vi "Advanced Cut - Main - Copy.vi"   [LabVIEW 2016] (continued)
"Desaccade"=FALSE, "Offset"=0.0, "Gain"=1.0}, {"Color"=16777224, "Visible"=TRUE, "Channel"=13, "Invert"=FALSE, "Desaccade"=FALSE, "Offset"=0.0, "Gain"=1.0}, {"Color"=16777224, "Visible"=FALSE, "Channel"=14, "Invert"=FALSE, "Desaccade"=FALSE, "Offset"=0.0, "Gain"=1.0}, {"Color"=16777224, "Visible"=FALSE, "Channel"=15, "Invert"=FALSE, "Desaccade"=FALSE, "Offset"=0.0, "Gain"=1.0}], "Experiment Parameters"={"Freq"=0.0, "Vel"=0, "Acc"=0, "Stimulus"="Head Impulse"}, "Autosort File"=refnum, "Data File"={"Data Channels"=array34x71049[2415666 elements], "Sample Rate"=500, "Channel List"=["Hz Position-in-Head", "Hz Velocity-in-Head", "Hy Position-in-Head", "Hy Velocity-in-Head", "Hx Position-in-Head", "Hx Velocity-in-Head", "Hl Velocity-in-Head", "Hr Velocity-in-Head", "Lx Position-in-Head", "Ly Position-in-Head", "Lz Position-in-Head", "Lx Velocity-in-Head", "Ly Velocity-in-Head", "Lz Velocity-in-Head", "Ll Velocity-in-Head", "Lr Velocity-in-Head", "Rx Position-in-Head", "Ry Position-in-Head", "Rz Position-in-Head", "Rx Velocity-in-Head", "Ry Velocity-in-Head", "Rz Velocity-in-Head", "Rl Velocity-in-Head", "Rr Velocity-in-Head", "Target on/off", "aux input 1", "aux input 2", " ", "", "", "", "Target Hor", "Target Ver", ""]}, "Experiment data path"=path "C:/Users/w.figtree/Desktop/Coils Data/3", "Image data path"=path "/Macintosh HD/Users/patrick/Studium/Diploma Thesis/Data Analysis", "LVS data path"=path "/Macintosh HD/Users/patrick/Studium/Diploma Thesis/Data Analysis", "Raw copy path"=path "/Macintosh HD/Users/patrick/Studium/Diploma Thesis/Data Analysis", "filename"="passive_lvs.lvs", "desaccading parameters"={"Tolerance"=3, "Acc Range"=7000.0, "Sample Rate"=500, "Impulse Plane 2"=enum."Yaw", "Impulse dir"=FALSE}, "Experiment Parameters 2"={"Subject"="SE Trial Short Term", "Strain"="", "Rotation plane"="", "Experimenter"=" ", "Trial"=0.0, "Time"=0.0}, "Excel"={"Excel._Application"=refnum, "Use Excel"=TRUE, "Worksheet SINE"=refnum, "Row SINE"=0, "Worksheet TRANS"=refnum, "Row TRANS"=0}, "Session Config File"=refnum, "Autosort Parameter Set"=4, "EMA Version"="EMA 2016a", "desacc "={"Threshold 1 [Acc]"=7000.0, "Threshold 2 [% of TH1]"=60, "tolerance"=3, "Search WD "=0.1, " always use TH2"=FALSE, "Range"=3.0, "Max time"=120.0, "Min time"=20.0, "Velocity Threshold"=150}, "Cycle Nr for Saccades"={"POS"=0, "NEG"=0}, "Undo Counter"=0, "History Length"=0, "Redo Counter"=0, "Histpry Position"=-1, "Raw Data File"={"Data Channels"=[], "Sample Rate"=0, "Channel List"=[]}, "calibration name"="u_calibration_1_p00001s001_calib.mat"} {"Parameter Time Series"."time offset" format="%.3f"; "Parameter Time Series"."Gain" format="%.1f"; "Parameter Time Series"."Offset" format="%.1f"; "Parameter Time Series"."List 1" items=["Motor-Pos", "Motor-Vel", "Lx Position-in-Head", "Ly Position-in-Head", "Lz Position-in-Head", "Lx Velocity-in-Head", "Ly Velocity-in-Head", "Lz Velocity-in-Head", "Ll Velocity-in-Head", "Lr Velocity-in-Head", "Lx Accel-in-Head", "Ly Accel-in-Head", "Lz Accel-in-Head", "Rx Position-in-Head", "Ry Position-in-Head", "Rz Position-in-Head", "Rx Velocity-in-Head", "Ry Velocity-in-Head", "Rz Velocity-in-Head", "Rl Velocity-in-Head", "Rr Velocity-in-Head", "Rx Accel-in-Head", "Ry Accel-in-Head", "Rz Accel-in-Head", "Global Trigger", "", "", ""]; "Parameter Impuls Series"."Gain" format="%.1f"; "Parameter Impuls Series"."Offset" format="%.1f"})   [LabVIEW 2016]
uses:
  Type Definitions/Advanced Cut States.ctl
  Type Definitions/Snippet.ctl
  <userlib>/_OpenG.lib/file/file.llb/Strip Path Extension - Path__ogtk.vi
  core/type-defs/TD_Impulse Parameter.ctl
  core/core.lvlib
  core/type-defs/TD_Time Series.ctl
  core/type-defs/TD_Statemachine-Data.ctl
panel:
  out "Time Series Graph":cluster{"Ramp Pattern":dbl[], dbl[]}[](graph)
  in  "Snippet File Suffix":string
  in  "btn_DoCut":bool
  in  "btn_AutoSnippet":bool
  in  "btn_ClearTable":bool
  in  "Auto Snippet Options":T1
  in  "Snippet Table":string[][](table)
  in  "Parameter Time Series":T5(array[cluster]) caption="X-off    Y-off     Gain   Inv Filt Dot Int                      Channel                                  Vis" {"time offset" format="%.3f"; "Gain" format="%.1f"; "Offset" format="%.1f"; "List 1" items=["-", "Hz Velocity-in-Head", "-", "Hy Velocity-in-Head", "-", "Hx Velocity-in-Head", "Hl Velocity-in-Head", "Hr Velocity-in-Head", "-", "Ly Position-in-Head", "Lz Position-in-Head", "-", "Ly Velocity-in-Head", "Lz Velocity-in-Head", "-", "-", "-", "-", "-", "-", "-", "-", "-", "-"]}
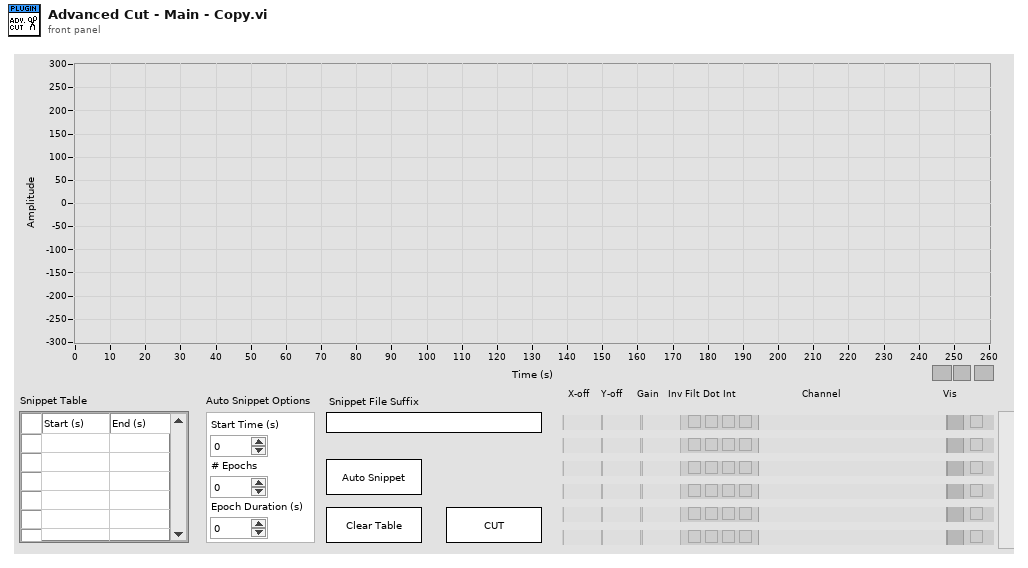
[diagram p1: front panel]
types:
  T1 = cluster{"Start Time (s)":dbl, "# Epochs":u32, "Epoch Duration (s)":dbl}
  T2 = typedef "core.lvlib/TD_Statemachine-Data.ctl" = cluster{"Impulse Positions":cluster{"Start":i32, "End":i32, "Impulse Plane":enum16{"Other", "Yaw", "Pitch", "Roll", "LARP", "RALP"}, "Impulse Direction +ve?":bool, "Time offset":i32, "Amplitude offset":dbl}[], "Old Impulse positions for Undo":cluster{"Start":i32, "End":i32, "Impulse Plane":enum16{"Other", "Yaw", "Pitch", "Roll", "LARP", "RALP"}, "Impulse Direction +ve?":bool, "Time offset":i32, "Amplitude offset":dbl}[][], "No. Imp":i32, "Parameter Time Series":T3, "Parameter Impuls Series":T4, "Experiment Parameters":cluster{"Freq":dbl, "Vel":i32, "Acc":i32, "Stimulus":string}, "Autosort File":refnum<file>, "Data File":cluster{"Data Channels":dbl[][], "Sample Rate":i32, "Channel List":string[]}, "Experiment data path":path, "Image data path":path, "LVS data path":path, "Raw copy path":path, "filename":string, "desaccading parameters":cluster{"Tolerance":i32, "Acc Range":dbl, "Sample Rate":i32, "Impulse Plane 2":enum16{"Other", "Yaw", "Pitch", "Roll", "LARP", "RALP"}, "Impulse dir":bool}, "Experiment Parameters 2":cluster{"Subject":string, "Strain":string, "Rotation plane":string, "Experimenter":string, "Trial":dbl, "Time":dbl}, "Excel":cluster{"Excel._Application":refnum<k7>, "Use Excel":bool, "Worksheet SINE":refnum<k7>, "Row SINE":i32, "Worksheet TRANS":refnum<k7>, "Row TRANS":i32}, "Session Config File":refnum<file>, "Autosort Parameter Set":i32, "EMA Version":string, "desacc ":cluster{"Threshold 1 [Acc]":dbl, "Threshold 2 [% of TH1]":i32, "tolerance":i32, "Search WD ":dbl, " always use TH2":bool, "Range":dbl, "Max time":dbl, "Min time":dbl, "Velocity Threshold":i32}, "Cycle Nr for Saccades":cluster{"POS":i32, "NEG":i32}, "Undo Counter":i32, "History Length":i32, "Redo Counter":i32, "Histpry Position":i32, "Raw Data File":cluster{"Data Channels":dbl[][], "Sample Rate":i32, "Channel List":string[]}, "calibration name":string}
  T3 = typedef "core.lvlib/TD_Time Series.ctl" = cluster{"time offset":dbl, "Offset":dbl, "Gain":dbl, "inverse":bool, "filter data":bool, "dots":bool, "interpolate":bool, "List 1":u16, "Color Box":u32, "Boolean":bool}[]
  T4 = typedef "core.lvlib/TD_Impulse Parameter.ctl" = cluster{"Color":u32, "Visible":bool, "Channel":u16, "Invert":bool, "Desaccade":bool, "Offset":dbl, "Gain":dbl}[]
  T5 = cluster{"time offset":dbl, "Offset":dbl, "Gain":dbl, "inverse":bool, "filter data":bool, "dots":bool, "interpolate":bool, "List 1":u16, "Color Box":u32, "Boolean":bool}[]
  T6 = typedef "Snippet.ctl" = cluster{"Start Index":i32, "End Index":i32}
  T7 = typedef "Advanced Cut States.ctl" = enum16{"Initialise", "Quit", "DO Refresh Snippet Table", "DO Auto Snippet", "DO Clear Snippets", "DO Cut"}
  T8 = typedef "Advanced Cut States.ctl" = enum16{"Initialise", "Quit", "DO Draw", "Draw - Defer Updates", "Draw - Clear Time Series", "Draw - Time Series", "Draw - Snippet Table", "Draw - Enable Updates", "DO Auto Snippet", "DO Clear Snippets", "DO Cut"}
  T9 = cluster{"Data Channels":dbl[][], "Sample Rate":i32, "Channel List":string[]}
  T10 = cluster{"Data File":cluster{"Data Channels":dbl[][], "Sample Rate":i32, "Channel List":string[]}, "Data IN":T2}
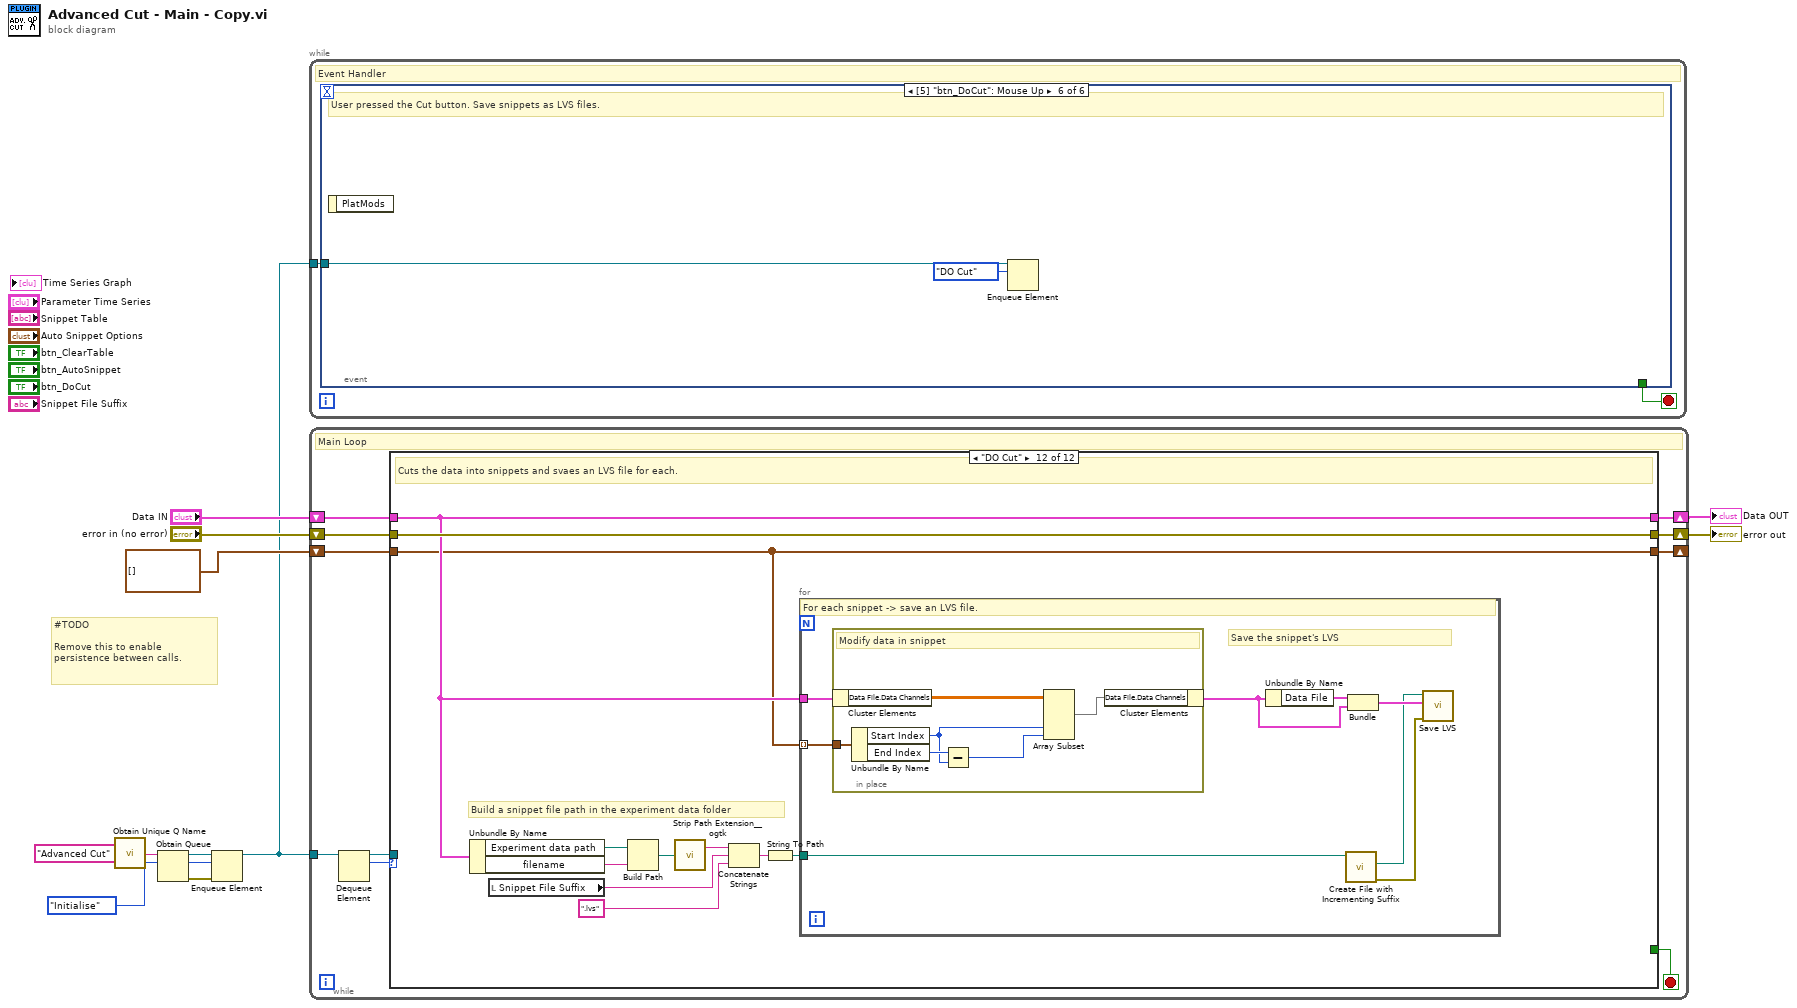
[diagram p0: block diagram]
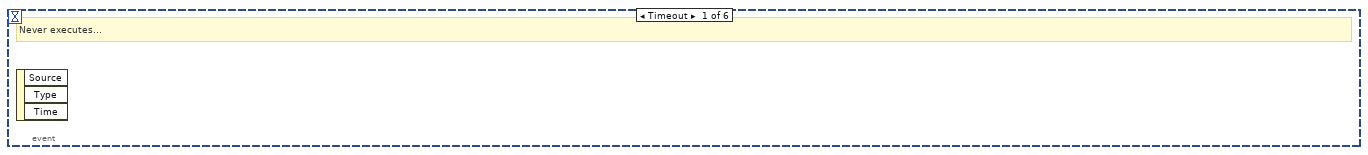
[diagram p2: hidden frame]
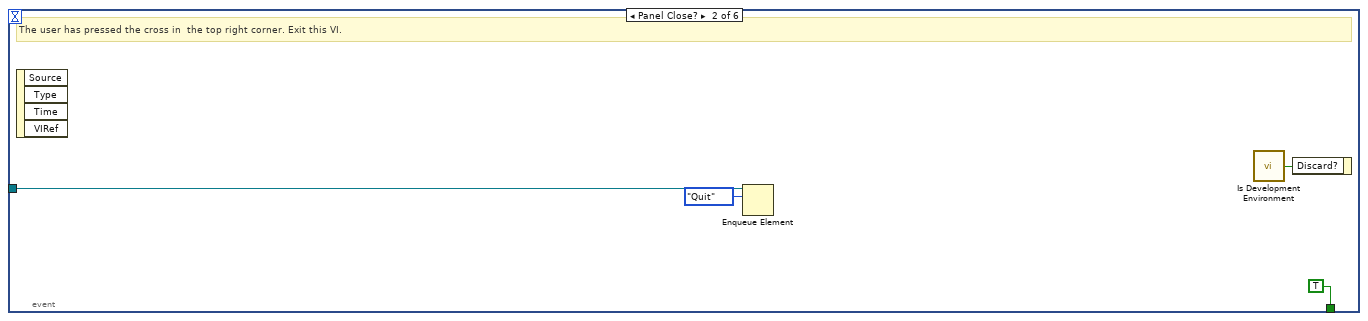
[diagram p3: hidden frame]
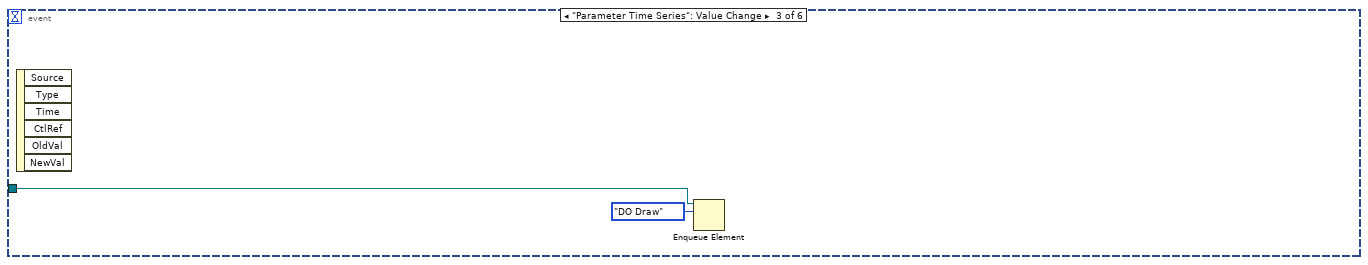
[diagram p4: hidden frame]
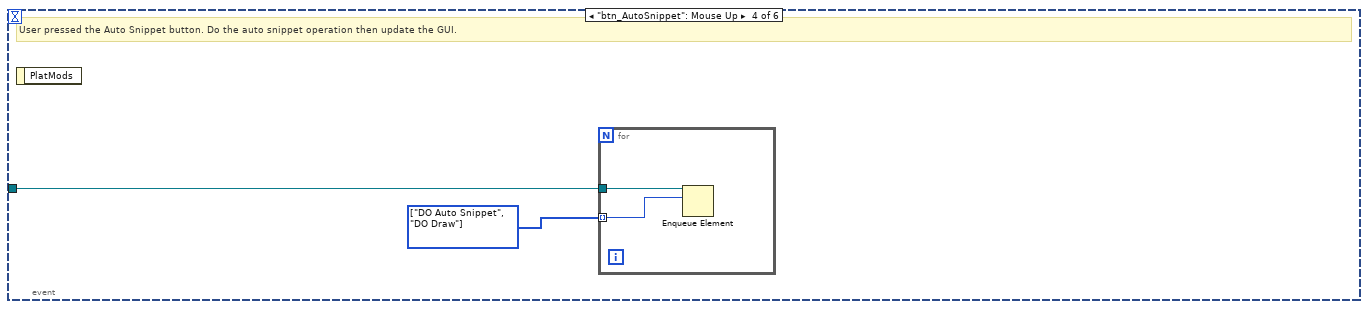
[diagram p5: hidden frame]
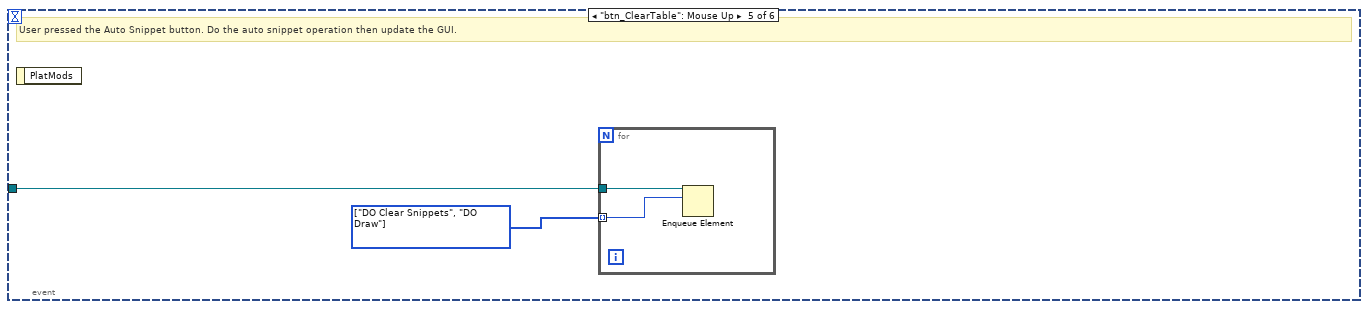
[diagram p6: hidden frame]
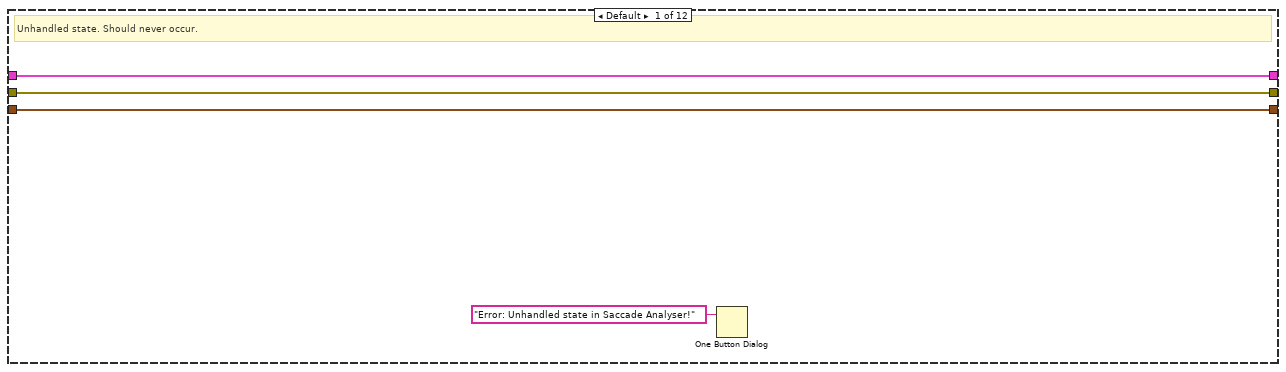
[diagram p7: hidden frame]
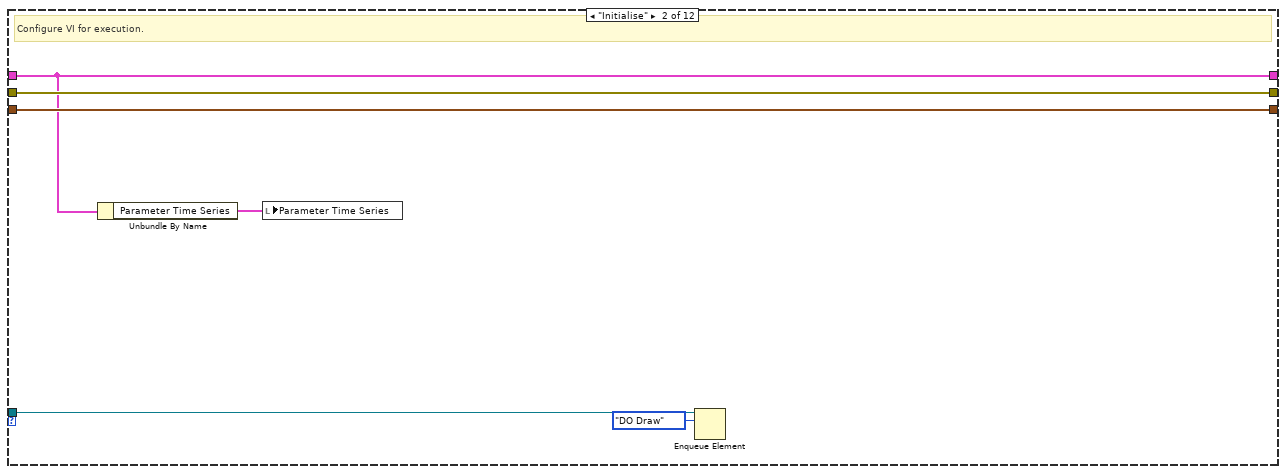
[diagram p8: hidden frame]
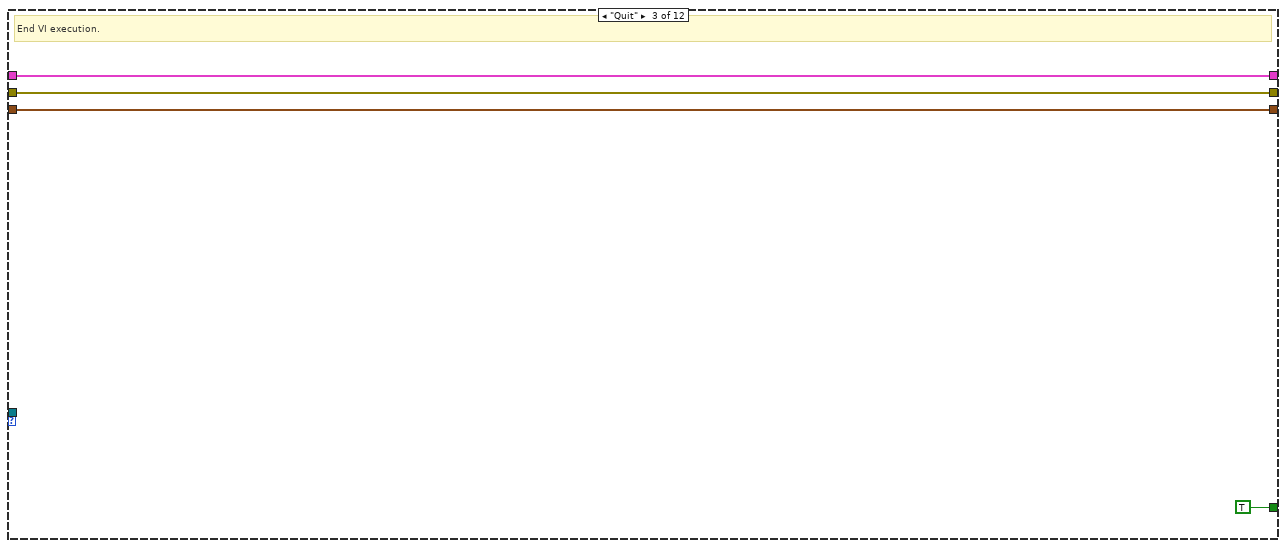
[diagram p9: hidden frame]
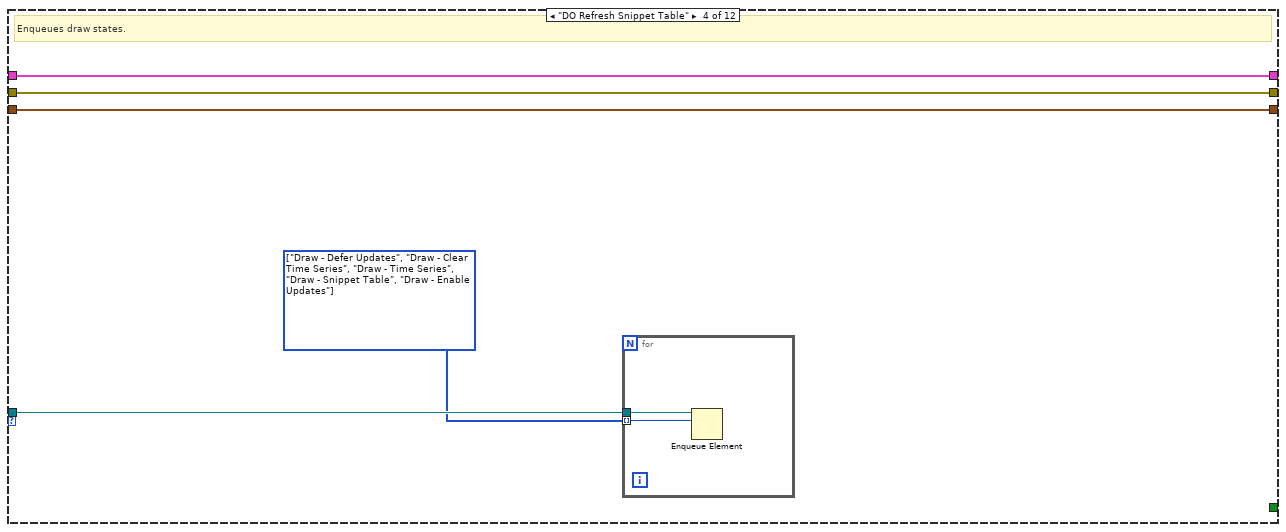
[diagram p10: hidden frame]
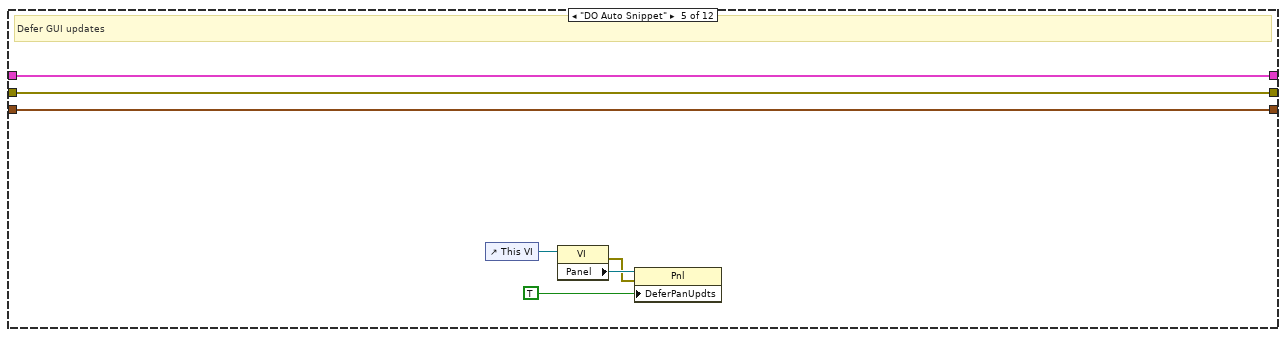
[diagram p11: hidden frame]
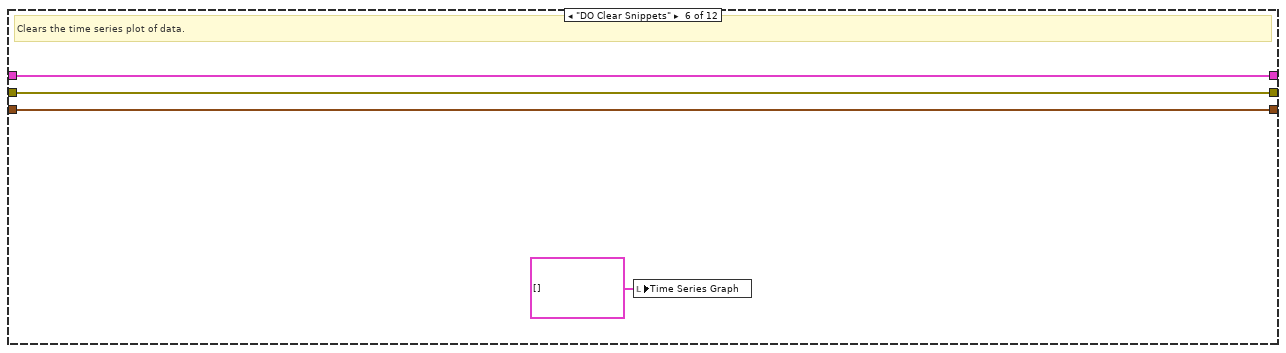
[diagram p12: hidden frame]
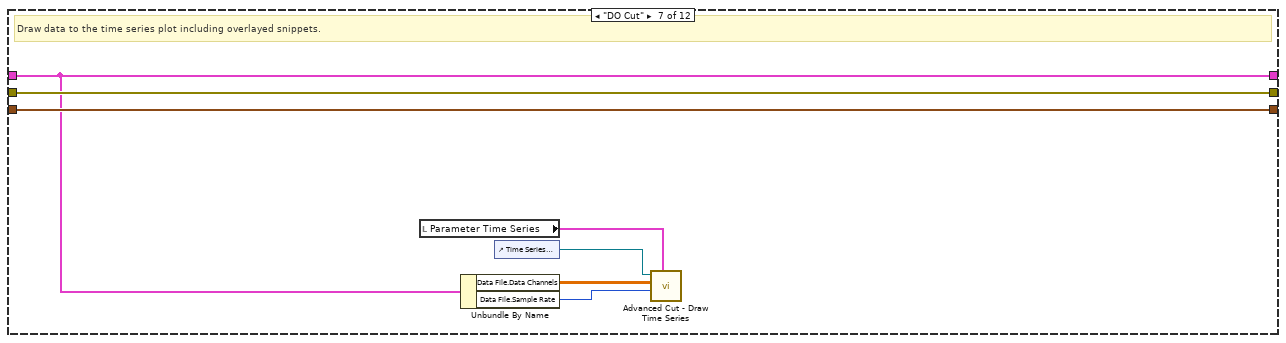
[diagram p13: hidden frame]
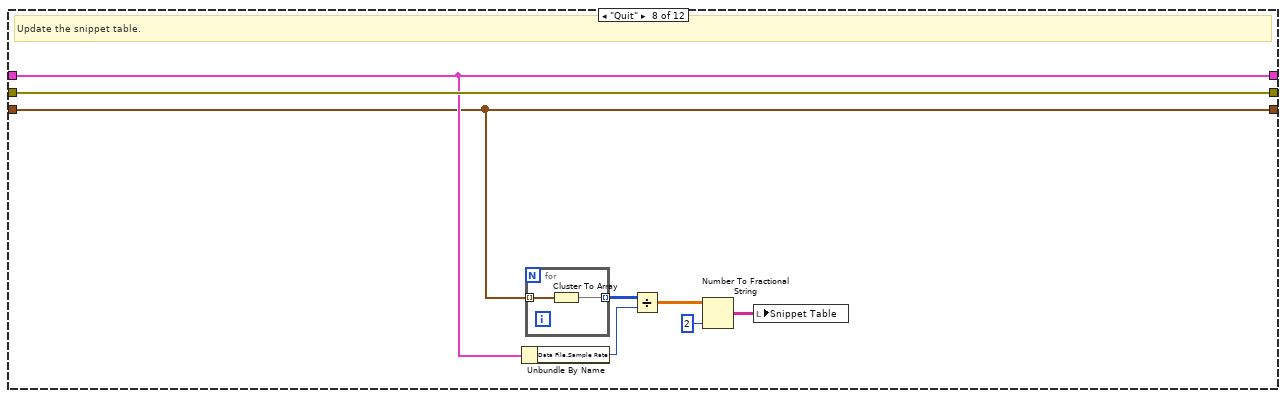
[diagram p14: hidden frame]
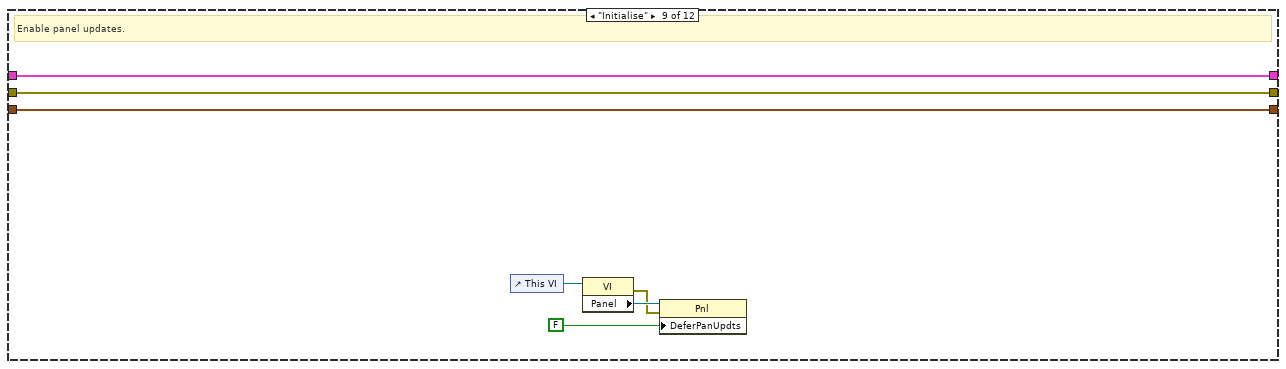
[diagram p15: hidden frame]
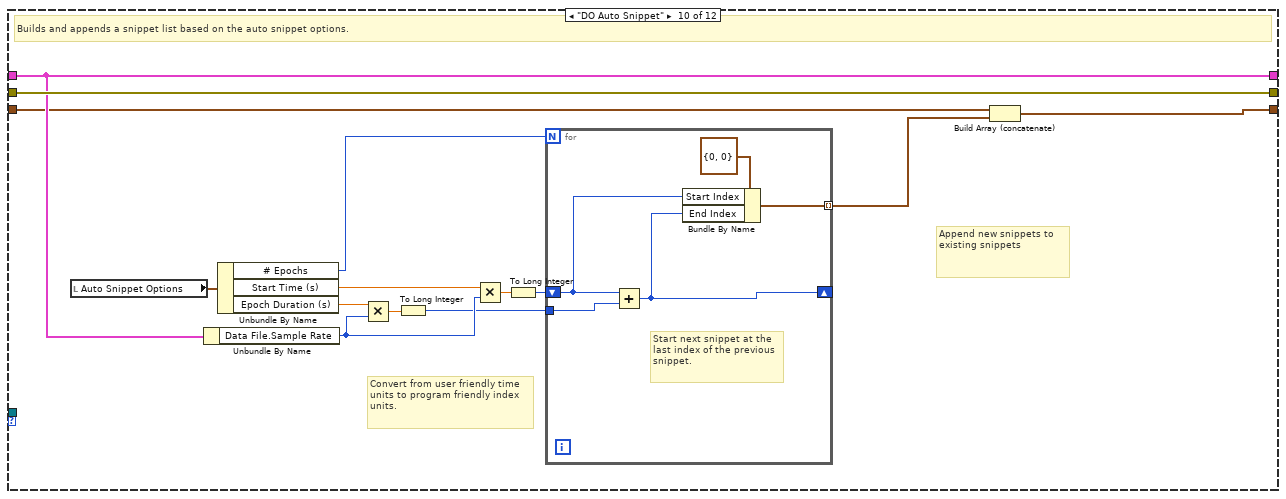
[diagram p16: hidden frame]
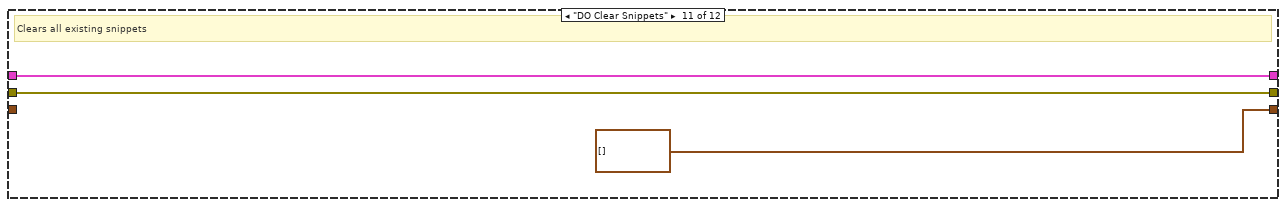
[diagram p17: hidden frame]
diagram:
  w3 = Advanced_Cut_States."Initialise" ("Advanced Cut States")
  # "#TODO\n\nRemove this to enable persistence between calls."
  n1 = call <userlib>:"Obtain Unique Q Name.vi"("Queue"="Advanced Cut") -> ("Q Name"=w4:string)  [unwired: 4 in]
  n2 = Obtain Queue(name (unnamed)=w4, element data type=w3) -> (queue out=w6:refnum<queue>, error out=w7:errorcluster)  [unwired: 3 in, 1 out]
  n3 = Enqueue Element(queue=w6, element=w3, error in (no error)=w7) -> (queue out=w1:refnum<queue>)  [unwired: 1 in, 2 out]
  n4 = while {
    tunnel: w1 -> [w12]
    stop <- w13 stop-if-true
    # "Event Handler"
    n5 = event shown="[5] \"btn_DoCut\": Mouse Up" {
      selector: _ -> [_ _ _ _ _ _]
      dyn-events: _ -> [_ _ _ _ _ _]
      timeout: _ -> [_ _ _ _ _ _]
      tunnel: [_ TRUE _ _ _ _] -> w13
      tunnel: w12 -> [_ w15 w18 w21 w25 w29]
      event Timeout {
        # "Never executes..."
        n6 = event-data() -> ()  [unwired: 1 in, 3 out]
      }
      event Panel Close? {
        # "The user has pressed the cross in  the top right corner. Exit this VI."
        n7 = event-data() -> ()  [unwired: 1 in, 4 out]
        n8 = Enqueue Element(queue=w15, element=Advanced_Cut_States."Quit") -> ()  [unwired: 2 in, 3 out]
        n9 = call <userlib>:"Is Development Environment.vi"() -> ("dev?"=w17:bool)
        n10 = event-data("Discard?"=w17) -> ()  [unwired: 1 in, 1 out]
      }
      event "Parameter Time Series": Value Change {
        n11 = event-data() -> ()  [unwired: 1 in, 6 out]
        n12 = Enqueue Element(queue=w18, element=Advanced_Cut_States."DO Draw") -> ()  [unwired: 2 in, 3 out]
      }
      event "btn_AutoSnippet": Mouse Up {
        w20 = T8[] [enum."DO Auto Snippet", enum."DO Draw"] items=["Initialise", "Quit", "DO Draw", "Draw - Defer Updates", "Draw - Clear Time Series", "Draw - Time Series", "Draw - Snippet Table", "Draw - Enable Updates", "DO Auto Snippet", "DO Clear Snippets", "DO Cut"] ("element")
        # "User pressed the Auto Snippet button. Do the auto snippet operation then update the GUI."
        n13 = event-data() -> ()  [unwired: 1 in, 1 out]
        n14 = for {
          tunnel: w21 -> [w23]
          tunnel: w20 -> [w22] mode=indexing
          n15 = Enqueue Element(queue=w23, element=w22) -> ()  [unwired: 2 in, 3 out]
        }
      }
      event "btn_ClearTable": Mouse Up {
        w24 = T8[] [enum."DO Clear Snippets", enum."DO Draw"] items=["Initialise", "Quit", "DO Draw", "Draw - Defer Updates", "Draw - Clear Time Series", "Draw - Time Series", "Draw - Snippet Table", "Draw - Enable Updates", "DO Auto Snippet", "DO Clear Snippets", "DO Cut"] ("element")
        # "User pressed the Auto Snippet button. Do the auto snippet operation then update the GUI."
        n16 = event-data() -> ()  [unwired: 1 in, 1 out]
        n17 = for {
          tunnel: w25 -> [w27]
          tunnel: w24 -> [w26] mode=indexing
          n18 = Enqueue Element(queue=w27, element=w26) -> ()  [unwired: 2 in, 3 out]
        }
      }
      event "btn_DoCut": Mouse Up {
        # "User pressed the Cut button. Save snippets as LVS files."
        n19 = event-data() -> ()  [unwired: 1 in, 1 out]
        n20 = Enqueue Element(queue=w29, element=Advanced_Cut_States."DO Cut") -> ()  [unwired: 2 in, 3 out]
      }
    }
  }
  n21 = while {
    shift-right: [w36] -> w9
    shift-left: "Data IN" -> [w37]
    shift-right: [w34] -> w8
    shift-left: "error in (no error)" -> [w35]
    tunnel: w1 -> [w39]
    shift-right: [w31] -> _
    shift-left: T6[] [] ("Array") -> [w32]
    stop <- w33 stop-if-true
    # "Main Loop"
    n22 = Dequeue Element(queue=w39) -> (queue out=w30:refnum<queue>, element=w38:T7)  [unwired: 2 in, 2 out]
    n23 = case shown="\"DO Cut\"" w38 {
      tunnel: w37 -> [w42 w45 w53 w58 w67 w71 w76 w85 w95 w107 w116 w127]
      tunnel: [w42 w45 w53 w58 w67 w71 w76 w85 w95 w107 w116 w127] -> w36
      tunnel: w35 -> [w41 w49 w52 w57 w66 w70 w78 w86 w94 w109 w117 w128]
      tunnel: [w41 w49 w52 w57 w66 w70 w78 w86 w94 w109 w117 w128] -> w34
      tunnel: [_ _ TRUE _ _ _ _ _ _ _ _ _] -> w33
      tunnel: w32 -> [w40 w48 w50 w56 w65 w69 w77 w79 w93 w98 _ w123]
      tunnel: [w40 w48 w50 w56 w65 w69 w77 w79 w93 w97 T6[] [] ("Array") w123] -> w31
      tunnel: w30 -> [_ w47 _ w55 _ _ _ _ _ _ _ _]
      frame Default {
        # "Unhandled state. Should never occur."
        n24 = One Button Dialog(message="Error: Unhandled state in Saccade Analyser!") -> ()  [unwired: 1 in, 1 out]
      }
      frame "Initialise" {
        # "Configure VI for execution."
        n25 = Unbundle By Name(w45) -> ("Parameter Time Series"=w44:T3)
        n26 = local write "Parameter Time Series"(w44) -> ()
        n27 = Enqueue Element(queue=w47, element=Advanced_Cut_States."DO Draw") -> ()  [unwired: 2 in, 3 out]
      }
      frame "Quit" {
        # "End VI execution."
      }
      frame "DO Refresh Snippet Table" {
        w54 = T8[] [enum."Draw - Defer Updates", enum."Draw - Clear Time Series", enum."Draw - Time Series", enum."Draw - Snippet Table", enum."Draw - Enable Updates"] items=["Initialise", "Quit", "DO Draw", "Draw - Defer Updates", "Draw - Clear Time Series", "Draw - Time Series", "Draw - Snippet Table", "Draw - Enable Updates", "DO Auto Snippet", "DO Clear Snippets", "DO Cut"] ("Array")
        # "Enqueues draw states."
        n28 = for {
          tunnel: w55 -> [w60]
          tunnel: w54 -> [w59] mode=indexing
          n29 = Enqueue Element(queue=w60, element=w59) -> ()  [unwired: 2 in, 3 out]
        }
      }
      frame "DO Auto Snippet" {
        # "Defer GUI updates"
        n30 = control-ref of="This VI"() -> (w64:refnum<vi>)
        n31 = property class="VI"(reference=w64) -> (error out=w62:errorcluster, "Panel"=w63:refnum<vi>)  [unwired: 1 in, 1 out]
        n32 = property class="Pnl"(reference=w63, error in=w62, "DeferPanUpdts"=TRUE ("Defer Panel Updates")) -> ()  [unwired: 2 out]
      }
      frame "DO Clear Snippets" {
        # "Clears the time series plot of data."
        n33 = local write "Time Series Graph"(cluster{"Ramp Pattern":dbl[], dbl[]}[] [] ("Time Series Graph")) -> ()
      }
      frame "DO Cut" {
        # "Draw data to the time series plot including overlayed snippets."
        n34 = local read "Parameter Time Series"() -> (w73:T5)
        n35 = Unbundle By Name(w76) -> ("Data File.Data Channels"=w75:dbl[][], "Data File.Sample Rate"=w74:i32)
        n36 = control-ref of="Time Series Graph"() -> (w72:refnum<vi>)
        n37 = call "Advanced Cut - Draw Time Series.vi"("Parameter Time Series"=w73, "Sample Rate"=w74, "Data"=w75, "Time Series Graph in"=w72) -> ()  [unwired: 6 in, 2 out]
      }
      frame "Quit" {
        # "Update the snippet table."
        n38 = Unbundle By Name(w85) -> ("Data File.Sample Rate"=w83:i32)
        n39 = for {
          tunnel: w79 -> [w88] mode=indexing
          tunnel: [w87] -> w84 mode=indexing
          n40 = Cluster To Array(cluster=w88) -> (array=w87:i32[])
        }
        n41 = Divide(x=w84, y=w83) -> (x/y=w82:dbl[][])
        n42 = Number To Fractional String(number=w82, precision (6)=i16 2) -> (F-format string=w80:string[][])  [unwired: 2 in]
        n43 = local write "Snippet Table"(w80) -> ()
      }
      frame "Initialise" {
        # "Enable panel updates."
        n44 = control-ref of="This VI"() -> (w92:refnum<vi>)
        n45 = property class="VI"(reference=w92) -> (error out=w90:errorcluster, "Panel"=w91:refnum<vi>)  [unwired: 1 in, 1 out]
        n46 = property class="Pnl"(reference=w91, error in=w90, "DeferPanUpdts"=FALSE ("Defer Panel Updates")) -> ()  [unwired: 2 out]
      }
      frame "DO Auto Snippet" {
        # "Convert from user friendly time units to program friendly index units."
        # "Append new snippets to existing snippets"
        # "Builds and appends a snippet list based on the auto snippet options."
        n47 = local read "Auto Snippet Options"() -> (w108:T1)
        n48 = Unbundle By Name(w107) -> ("Data File.Sample Rate"=w104:i32)
        n49 = Unbundle By Name(w108) -> ("# Epochs"=w103:u32, "Start Time (s)"=w106:dbl, "Epoch Duration (s)"=w105:dbl)
        n50 = Multiply(x=w105, y=w104) -> (x*y=w100:dbl)
        n51 = To Long Integer(number=w100) -> (32bit integer=w99:i32)
        n52 = Multiply(x=w106, y=w104) -> (x*y=w102:dbl)
        n53 = To Long Integer(number=w102) -> (32bit integer=w101:i32)
        n54 = for {
          N: w103 -> [_]
          tunnel: w99 -> [w111]
          tunnel: [w113] -> w96 mode=indexing
          shift-right: [w110] -> _
          shift-left: w101 -> [w112]
          # "Start next snippet at the last index of the previous snippet."
          n55 = Add(x=w112, y=w111) -> (x+y=w110:i32)
          n56 = Bundle By Name(cluster=T6 {"Start Index"=0, "End Index"=0} ("Section"), "Start Index"=w112, "End Index"=w110) -> (w113:T6)
        }
        n57 = Build Array (concatenate)(w98, w96) -> (w97:T6[])
      }
      frame "DO Clear Snippets" {
        # "Clears all existing snippets"
      }
      frame "DO Cut" {
        # "Build a snippet file path in the experiment data folder"
        # "Cuts the data into snippets and svaes an LVS file for each."
        n58 = Unbundle By Name(w127) -> ("Experiment data path"=w126:path, "filename"=w125:string)
        n59 = local read "Snippet File Suffix"() -> (w121:string)
        n60 = Build Path(base path=w126, name or relative path=w125) -> (appended path=w124:path)
        n61 = call-poly <userlib>:"Strip Path Extension__ogtk.vi"("path"=w124) -> ("root"=w122:string)  [unwired: 1 out]
        n62 = Concatenate Strings(w122, w121, ".lvs") -> (w119:string)
        n63 = String To Path(string=w119) -> (path=w118:path)
        n64 = for {
          tunnel: w127 -> [w132]
          tunnel: w118 -> [w135]
          tunnel: w123 -> [w131] mode=indexing
          # "Save the snippet's LVS"
          # "For each snippet -> save an LVS file."
          n65 = in-place {
            in-place-border: w131 -> [w140]
            # "Modify data in snippet"
            n66 = in-place-cluster #1(w132) -> ("Data File.Data Channels"=w142:dbl[][])
            n67 = Unbundle By Name(w140) -> ("Start Index"=w137:i32, "End Index"=w139:i32)
            n68 = Subtract(x=w139, y=w137) -> (x-y=w138:i32)
            n69 = Array Subset(array=w142, index (col)=w137, length (col)=w138) -> (w141:dbl[][])  [unwired: 2 in]
            n70 = in-place-cluster #1("Data File.Data Channels"=w141) -> (w129:T2)
          }
          n71 = Unbundle By Name(w129) -> ("Data File"=w130:T9)
          n72 = call <vilib>:"Create File with Incrementing Suffix.vi"("file path"=w135) -> ("error out"=w133:errorcluster, "actual path"=w134:path)  [unwired: 8 in, 1 out]
          n73 = Bundle("Data File"=w130, "Data IN"=w129) -> (w136:T10)  [unwired: 1 in]
          n74 = call "Save LVS.vi"("error in (no error)"=w133, "LVS Data"=w136, "Path (in)"=w134) -> ()  [unwired: 7 in, 2 out]
        }
      }
    }
  }
  "Data OUT" <- w9
  "error out" <- w8
